vi "Controle_Manip_Main_GUI_Backup2.vi"() -> ()   [LabVIEW 2019] (continued)
                                }
                              }
                              n869 = local read "MasterStop"() -> (w1062:bool)
                            }
                            "Array fPow" <- w1052
                            "Array fPow Pow" <- w1054
                            n870 = Transpose 2D Array(2D array=w1052) -> (transposed array=w1051:i32[][])
                            n871 = property on="CCD 2D Image Main" class="IntGraph (strict)"("Value"=w1051) -> ()  [unwired: 2 in, 2 out]
                          }
                          frame #3 {
                            # "end"
                            n872 = control-ref of="Acquire fPow"() -> (w1194:refnum<vi>)
                            n873 = control-ref of="N Step Power  Diode Current (A)"() -> (w1195:refnum<vi>)
                            n874 = control-ref of="End Power  Diod Current (A)"() -> (w1196:refnum<vi>)
                            n875 = control-ref of="Start Power Diod Current (A)"() -> (w1197:refnum<vi>)
                            n876 = property class="Bool (strict)"(reference=w1194, "Value"=FALSE) -> ()  [unwired: 1 in, 2 out]
                            n877 = control-ref of="Acquire fPow"() -> (w1201:refnum<vi>)
                            n878 = control-ref of="Save fPow"() -> (w1199:refnum<vi>)
                            n879 = Build Array(w1201, w1199, w1197, w1196, w1195) -> (w1200:refnum<vi>[])
                            n880 = call "Enable&Disable_Controls.vi"("Enum"=enum16{"Enabled", "Disabled", "Disabled&Grayed"}."Enabled", "References"=w1200) -> ()  [unwired: 1 in]
                            n881 = property on="Elapsed (s)" class="DigNum (strict)"("Visible"=FALSE) -> ()  [unwired: 2 in, 2 out]
                            n882 = local read "Auto< ?"() -> (w1189:bool)
                            n883 = control-ref of="Save fPow"() -> (w1191:refnum<vi>)
                            n884 = case shown="True" w1189 {
                              tunnel: [TRUE FALSE] -> w1188
                              frame False {
                              }
                              frame True {
                              }
                            }
                            n885 = control-ref of="MasterStop"() -> (w1186:refnum<vi>)
                            n886 = control-ref of="MasterPause"() -> (w1187:refnum<vi>)
                            n887 = control-ref of="ExperimentStopped?"() -> (w1185:refnum<vi>)
                            n888 = call "CheckStopAndReset.vi"("ExperimentStopped?"=w1185, "MasterStop"=w1186, "MasterPause"=w1187) -> ()
                            n889 = control-ref of="Acquire fPow"() -> (w1192:refnum<vi>)
                            n890 = property class="Bool (strict)"(reference=w1192, "Visible"=TRUE) -> ()  [unwired: 1 in, 2 out]
                            n891 = property class="Bool (strict)"(reference=w1191, "Visible"=w1188) -> ()  [unwired: 1 in, 2 out]
                            n892 = property on="CCD 2D Image Main" class="IntGraph (strict)"("Visible"=TRUE) -> ()  [unwired: 2 in, 2 out]
                            n893 = property on="CCD 1D Spectrum Main" class="XYGraph (strict)"("Visible"=FALSE) -> ()  [unwired: 2 in, 2 out]
                          }
                        }
                      }
                      frame "Fast Acq" {
                        n894 = stacked-sequence {
                          frame #0 {
                            w1204 = AcqMode."Spectrum" ("Acq Mode")
                            # "set port to CCD if not already"
                            n895 = property on="Acq Mode" class="Enum (strict)"() -> ("Value"=w1206:T3)  [unwired: 2 in, 2 out]
                            n896 = Not Equal?(x=w1206, y=w1204) -> (x != y?=w1205:bool)
                            n897 = case shown="True" w1205 {
                              tunnel: w1204 -> [_ w1208]
                              frame False {
                              }
                              frame True {
                                w1207 = T33 4 items=["None"=1, "SideEntrance"=2, "FrontEntrance"=3, "SideExit"=5, "FrontExit"=4] ("Exit Port Location")
                                n898 = local read "LightField Automation error out"() -> (w1218:errorcluster)
                                n899 = local read "LightField Automation out"() -> (w1217:refnum<class "LightField Automation.lvclass">)
                                n900 = property on="Acq Mode" class="Enum (strict)"("Value"=w1208) -> ()  [unwired: 2 in, 2 out]
                                n901 = call "spec_SetOpticalExitPort.vi"("error in (no error)"=w1218, "Exit Port Location"=w1207, "LightField Automation in"=w1217) -> ("error out"=w1210:errorcluster, "LightField Automation out"=w1209:refnum<class "LightField Automation.lvclass">)  [unwired: 7 in]
                                n902 = call "spec_GetCenterWavelength.vi"("error in (no error)"=w1210, "LightField Automation in"=w1209) -> ("error out"=w1213:errorcluster, "Center Wavelength"=w1211:dbl, "LightField Automation out"=w1212:refnum<class "LightField Automation.lvclass">)  [unwired: 7 in]
                                n903 = local write "Exit mirror"(w1207) -> ()
                                n904 = local write "Center Wavelength (nm)"(w1211) -> ()
                                n905 = call "spec_getCalibration.vi"("error in (no error)"=w1213, "LightField Automation in"=w1212) -> ("error out"=w1216:errorcluster, "ColumnCalibration"=w1214:dbl[], "LightField Automation out"=w1215:refnum<class "LightField Automation.lvclass">)  [unwired: 7 in]
                                n906 = local write "Wavelength calibration"(w1214) -> ()
                                n907 = local write "LightField Automation error out"(w1216) -> ()
                                n908 = local write "LightField Automation out"(w1215) -> ()
                              }
                            }
                          }
                          frame #1 {
                            # "background if none"
                            n909 = local read "Background taken?"() -> (w1219:bool)
                            n910 = case shown="False" w1219 {
                              frame False {
                                n911 = stacked-sequence {
                                tunnel: [_ _ w1265] -> w1220
                                frame #0 {
                                n912 = property on="CCD 1D Spectrum Main" class="XYGraph (strict)"("YScale.Offset"=0.0 ("Y Scale.Offset and Multiplier:Offset")) -> ()  [unwired: 2 in, 2 out]
                                }
                                frame #1 {
                                # "make sure shutter is closed"
                                n913 = local read "KCube Shutter On?"() -> (w1251:bool)
                                n914 = control-ref of="Shutter Ctrls"() -> (w1255:refnum<vi>)
                                n915 = property class="Ring (strict)"(reference=w1255) -> ("Value"=w1254:u16)  [unwired: 1 in, 2 out]
                                n916 = control-ref of="KCube Shutter Device Reference"() -> (w1256:refnum<vi>)
                                n917 = Equal?(x=w1254, y=u16 0) -> (x = y?=w1252:bool)
                                n918 = case shown="False" w1252 {
                                tunnel: w1256 -> [w1259 _]
                                tunnel: w1255 -> [w1258 _]
                                tunnel: w1251 -> [w1257 _]
                                frame False {
                                n919 = call "Shutter.vi"("KCube Shutter Device Reference 2"=w1259, "Shutter Ctrls 2"=w1258, "Shutter on?"=w1257) -> ()
                                }
                                frame True {
                                }
                                }
                                }
                                frame #2 {
                                # "acquire"
                                n920 = local read "LightField Automation error out"() -> (w1263:errorcluster)
                                n921 = local read "LightField Automation out"() -> (w1264:refnum<class "LightField Automation.lvclass">)
                                n922 = local read "Accumulations"() -> (w1260:dbl)
                                n923 = call "LFA_Capture.vi"("error in (no error)"=w1263, "Frames"=w1260, "LightField Automation in"=w1264) -> ("error out"=w1262:errorcluster, "Data"=w1265:T26, "LightField Automation out"=w1261:refnum<class "LightField Automation.lvclass">)  [unwired: 6 in]
                                n924 = local write "LightField Automation error out"(w1262) -> ()
                                n925 = local write "LightField Automation out"(w1261) -> ()
                                }
                                }
                                n926 = local read "Acq Mode"() -> (w1221:T3)
                                n927 = case shown="\"Spectrum\", Default" w1221 {
                                selector: w1221 -> [w1222 w1240]
                                tunnel: w1220 -> [w1223 w1241]
                                frame "Spectrum", Default {
                                n928 = stacked-sequence {
                                tunnel: w1223 -> [_ w1234 _ _]
                                tunnel: w1222 -> [_ w1232 _ _]
                                frame #0 {
                                n929 = property on="CCD 2D Image Main" class="IntGraph (strict)"("Visible"=FALSE) -> ()  [unwired: 2 in, 2 out]
                                n930 = property on="CCD 1D Spectrum Main" class="XYGraph (strict)"("Visible"=TRUE) -> ()  [unwired: 2 in, 2 out]
                                }
                                frame #1 {
                                n931 = local read "Wavelength calibration"() -> (w1231:dbl[])
                                n932 = local read "CCD ROI"() -> (w1227:T20)
                                n933 = Divide(x=1239.842, y=w1231) -> (x/y=w1229:dbl[])
                                n934 = call "PrepareData4Graph.vi"("Wavelength nm"=w1229, "DataLF"=w1234, "CCD ROI"=w1227, "AcqMode"=w1232, "Data type"=T30."Spectre") -> ("Spectrum"=w1233:cluster{"Array 2":dbl[], "Array":dbl[]}, "PLInt out"=w1226:dbl[])  [unwired: 2 in, 2 out]
                                n935 = local write "CCD 1D Spectrum Main"(w1233) -> ()
                                n936 = local write "BackgroundSpec"(w1226) -> ()
                                }
                                frame #2 {
                                n937 = local read "BackgroundSpec"() -> (w1235:dbl[])
                                n938 = call-poly <vilib>:"Mean.vi"("X"=w1235) -> ("mean"=w1237:dbl)  [unwired: 1 out]
                                n939 = Negate(x=w1237) -> (-x=w1236:dbl)
                                n940 = property on="CCD 1D Spectrum Main" class="XYGraph (strict)"("YScale.Offset"=w1236) -> ()  [unwired: 2 in, 2 out]
                                }
                                frame #3 {
                                n941 = local write "Background taken?"(TRUE ("Background taken?")) -> ()
                                n942 = property on="Background substract" class="Enum (strict)"("Value"=enum16{"None", "Shutter"}."None" ("Background substract")) -> ()  [unwired: 2 in, 2 out]
                                }
                                }
                                }
                                frame "Image" {
                                n943 = stacked-sequence {
                                tunnel: w1241 -> [_ w1249]
                                tunnel: w1240 -> [_ w1247]
                                frame #0 {
                                n944 = property on="CCD 1D Spectrum Main" class="XYGraph (strict)"("Visible"=FALSE) -> ()  [unwired: 2 in, 2 out]
                                n945 = property on="CCD 2D Image Main" class="IntGraph (strict)"("Visible"=TRUE) -> ()  [unwired: 2 in, 2 out]
                                }
                                frame #1 {
                                n946 = local read "Wavelength calibration"() -> (w1248:dbl[])
                                n947 = local read "CCD ROI"() -> (w1244:T20)
                                n948 = call "PrepareData4Graph.vi"("Wavelength nm"=w1248, "DataLF"=w1249, "CCD ROI"=w1244, "AcqMode"=w1247, "Data type"=T30."Spectre") -> ("Intensity Graph"=w1246:dbl[][])  [unwired: 2 in, 3 out]
                                n949 = local write "CCD 2D Image Main"(w1246) -> ()
                                }
                                }
                                }
                                }
                              }
                              frame True {
                              }
                            }
                          }
                          frame #2 {
                            # "\"measurement\""
                            n950 = stacked-sequence {
                              frame #0 {
                                # "open shutter if closed"
                                n951 = control-ref of="Shutter Ctrls"() -> (w1267:refnum<vi>)
                                n952 = property class="Ring (strict)"(reference=w1267) -> ("Value"=w1269:u16)  [unwired: 1 in, 2 out]
                                n953 = local read "KCube Shutter On?"() -> (w1272:bool)
                                n954 = control-ref of="KCube Shutter Device Reference"() -> (w1268:refnum<vi>)
                                n955 = property on="Experiment Graph Controls" class="TabCtl (strict)"("Value"=T25."Spectrum" ("Experiment Graph Controls")) -> ()  [unwired: 2 in, 2 out]
                                n956 = Equal?(x=w1269, y=u16 0) -> (x = y?=w1271:bool)
                                n957 = case shown="True" w1271 {
                                tunnel: w1268 -> [_ w1275]
                                tunnel: w1267 -> [_ w1274]
                                tunnel: w1272 -> [_ w1273]
                                frame False {
                                }
                                frame True {
                                n958 = call "Shutter.vi"("KCube Shutter Device Reference 2"=w1275, "Shutter Ctrls 2"=w1274, "Shutter on?"=w1273) -> ()
                                }
                                }
                              }
                              frame #1 {
                                # "set CCD ROI and acquire"
                                n959 = local read "LightField Automation error out"() -> (w1283:errorcluster)
                                n960 = local read "LightField Automation out"() -> (w1284:refnum<class "LightField Automation.lvclass">)
                                n961 = local read "CCD ROI"() -> (w1282:T20)
                                n962 = local read "Accumulations"() -> (w1279:dbl)
                                n963 = call "Adv_SetROI.vi"("error in (no error)"=w1283, "ROI"=w1282, "LightField Automation in"=w1284) -> ("error out"=w1280:errorcluster, "LightField Automation out"=w1281:refnum<class "LightField Automation.lvclass">)  [unwired: 7 in]
                                n964 = call "LFA_Capture.vi"("error in (no error)"=w1280, "Frames"=w1279, "LightField Automation in"=w1281) -> ("error out"=w1277:errorcluster, "Data"=w1276:T26, "LightField Automation out"=w1278:refnum<class "LightField Automation.lvclass">)  [unwired: 6 in]
                                n965 = local write "LightField Automation out"(w1278) -> ()
                                n966 = local write "LightField Automation error out"(w1277) -> ()
                                n967 = local write "Data"(w1276) -> ()
                              }
                              frame #2 {
                                # "close shutter"
                                n968 = local read "KCube Shutter On?"() -> (w1287:bool)
                                n969 = control-ref of="KCube Shutter Device Reference"() -> (w1286:refnum<vi>)
                                n970 = control-ref of="Shutter Ctrls"() -> (w1285:refnum<vi>)
                                n971 = call "Shutter.vi"("KCube Shutter Device Reference 2"=w1286, "Shutter Ctrls 2"=w1285, "Shutter on?"=w1287) -> ()
                              }
                              frame #3 {
                                # "Show data accordingly"
                                n972 = local read "Acq Mode"() -> (w1289:T3)
                                n973 = local read "Data"() -> (w1288:T26)
                                n974 = case shown="\"Spectrum\", Default" w1289 {
                                selector: w1289 -> [w1290 w1309]
                                tunnel: w1288 -> [w1291 w1310]
                                frame "Spectrum", Default {
                                n975 = stacked-sequence {
                                tunnel: w1291 -> [_ w1307 _]
                                tunnel: w1290 -> [_ w1305 _]
                                frame #0 {
                                n976 = property on="CCD 1D Spectrum Main" class="XYGraph (strict)"("Visible"=TRUE) -> ()  [unwired: 2 in, 2 out]
                                n977 = property on="CCD 2D Image Main" class="IntGraph (strict)"("Visible"=FALSE) -> ()  [unwired: 2 in, 2 out]
                                }
                                frame #1 {
                                n978 = local read "Wavelength calibration"() -> (w1304:dbl[])
                                n979 = local read "CCD ROI"() -> (w1300:T20)
                                n980 = Divide(x=1239.842, y=w1304) -> (x/y=w1302:dbl[])
                                n981 = call "PrepareData4Graph.vi"("Wavelength nm"=w1302, "DataLF"=w1307, "CCD ROI"=w1300, "AcqMode"=w1305, "Data type"=T30."Spectre") -> ("Spectrum"=w1306:cluster{"Array 2":dbl[], "Array":dbl[]}, "PLInt out"=w1299:dbl[])  [unwired: 2 in, 2 out]
                                n982 = local read "Excitation Power (uW)"() -> (w1296:dbl)
                                n983 = local write "CCD 1D Spectrum Main"(w1306) -> ()
                                n984 = local read "Acq Time (ms)"() -> (w1297:dbl)
                                n985 = local read "BackgroundSpec"() -> (w1295:dbl[])
                                n986 = local read "Display Mode"() -> (w1294:u16)
                                n987 = control-ref of="Cnts"() -> (w1298:refnum<vi>)
                                n988 = call "2Cnts.vi"("Array Background"=w1295, "Pow W"=w1296, "AcqTime ms"=w1297, "Cnts Ref"=w1298, "Display Mode"=w1294, "Array"=w1299) -> ()  [unwired: 1 out]
                                }
                                frame #2 {
                                n989 = property on="Full scale" class="Bool (strict)"("Val(Sgnl)"=TRUE ("Value (Signaling)")) -> ()  [unwired: 2 in, 2 out]
                                }
                                }
                                }
                                frame "Image" {
                                n990 = stacked-sequence {
                                tunnel: w1310 -> [_ w1318]
                                tunnel: w1309 -> [_ w1316]
                                frame #0 {
                                n991 = property on="CCD 1D Spectrum Main" class="XYGraph (strict)"("Visible"=FALSE) -> ()  [unwired: 2 in, 2 out]
                                n992 = property on="CCD 2D Image Main" class="IntGraph (strict)"("Visible"=TRUE) -> ()  [unwired: 2 in, 2 out]
                                }
                                frame #1 {
                                n993 = local read "Wavelength calibration"() -> (w1317:dbl[])
                                n994 = local read "CCD ROI"() -> (w1313:T20)
                                n995 = call "PrepareData4Graph.vi"("Wavelength nm"=w1317, "DataLF"=w1318, "CCD ROI"=w1313, "AcqMode"=w1316, "Data type"=T30."Spectre") -> ("Intensity Graph"=w1315:dbl[][])  [unwired: 2 in, 3 out]
                                n996 = local write "CCD 2D Image Main"(w1315) -> ()
                                }
                                }
                                }
                                }
                              }
                            }
                          }
                        }
                      }
                      frame "Acquire Custom Diode Spectrum" {
                        n997 = stacked-sequence {
                          frame #0 {
                            # "change exit slit to APD if needed"
                            n998 = local read "Spectrum Custom Mode"() -> (w1320:u16)
                            n999 = case shown="3" w1320 {
                              frame 0, Default {
                                n1000 = control-ref of="Accumulations"() -> (w1327:refnum<vi>)
                                n1001 = control-ref of="CCD ROI"() -> (w1328:refnum<vi>)
                                n1002 = control-ref of="Exposure Time (ms)"() -> (w1329:refnum<vi>)
                                n1003 = stacked-sequence {
                                tunnel: u16 5 ("NewVal") -> [w1331 w1336 _]
                                tunnel: [_ w1335 _] -> w1325
                                tunnel: [_ w1334 _] -> w1324
                                frame #0 {
                                n1004 = control-ref of="Exit mirror"() -> (w1330:refnum<vi>)
                                n1005 = property class="Ring (strict)"(reference=w1330, "Value"=w1331) -> ()  [unwired: 1 in, 2 out]
                                n1006 = Build Array(w1330) -> (w1333:refnum<vi>[])
                                n1007 = call "Enable&Disable_Controls.vi"("Enum"=enum16{"Enabled", "Disabled", "Disabled&Grayed"}."Disabled&Grayed", "References"=w1333) -> ()  [unwired: 1 in]
                                }
                                frame #1 {
                                n1008 = local read "LightField Automation error out"() -> (w1344:errorcluster)
                                n1009 = case shown="4, Default" w1336 {
                                tunnel: [enum16{"Enabled", "Disabled", "Disabled&Grayed"}."Disabled&Grayed" ("Enum") enum16{"Enabled", "Disabled", "Disabled&Grayed"}."Enabled" ("Enum")] -> w1335
                                tunnel: [AcqMode."APD 1" ("Acq Mode") AcqMode."Spectrum" ("Acq Mode")] -> w1334
                                frame 5 {
                                }
                                frame 4, Default {
                                }
                                }
                                n1010 = local read "LightField Automation out"() -> (w1343:refnum<class "LightField Automation.lvclass">)
                                n1011 = call "spec_GetOpticalExitPort.vi"("error in (no error)"=w1344, "LightField Automation in"=w1343) -> ("error out"=w1341:errorcluster, "Exit Port Location"=w1340:T33, "LightField Automation out"=w1342:refnum<class "LightField Automation.lvclass">)  [unwired: 7 in]
                                n1012 = Equal?(x=w1340, y=w1336) -> (x = y?=w1339:bool)
                                n1013 = case shown="False" w1339 {
                                tunnel: w1342 -> [w1365 w1367]
                                tunnel: w1341 -> [w1364 w1366]
                                tunnel: w1336 -> [w1363 _]
                                tunnel: [w1356 w1367] -> w1338
                                tunnel: [w1355 w1366] -> w1337
                                frame False {
                                n1014 = call "spec_SetOpticalExitPort.vi"("error in (no error)"=w1364, "Exit Port Location"=w1363, "LightField Automation in"=w1365) -> ("error out"=w1358:errorcluster, "LightField Automation out"=w1357:refnum<class "LightField Automation.lvclass">)  [unwired: 7 in]
                                n1015 = call "spec_GetCenterWavelength.vi"("error in (no error)"=w1358, "LightField Automation in"=w1357) -> ("error out"=w1361:errorcluster, "Center Wavelength"=w1359:dbl, "LightField Automation out"=w1360:refnum<class "LightField Automation.lvclass">)  [unwired: 7 in]
                                n1016 = local write "Center Wavelength (nm)"(w1359) -> ()
                                n1017 = call "spec_getCalibration.vi"("error in (no error)"=w1361, "LightField Automation in"=w1360) -> ("error out"=w1355:errorcluster, "ColumnCalibration"=w1362:dbl[], "LightField Automation out"=w1356:refnum<class "LightField Automation.lvclass">)  [unwired: 7 in]
                                n1018 = local write "Wavelength calibration"(w1362) -> ()
                                n1019 = property on="Exit mirror" class="Ring (strict)"() -> ("RingText.Text"=w1351:string)  [unwired: 2 in, 2 out]
                                n1020 = local read "Log file"() -> (w1354:string)
                                n1021 = Concatenate Strings("Exit mirror set to " ("Add to log file"), w1351) -> (w1352:string)
                                n1022 = call "Write2LogFile.vi"("Add to log file"=w1352, "Log file before"=w1354, "Checkbox"=FALSE) -> ("Log file after"=w1353:string)
                                n1023 = local write "Log file"(w1353) -> ()
                                }
                                frame True {
                                }
                                }
                                n1024 = local write "LightField Automation error out"(w1337) -> ()
                                n1025 = local write "LightField Automation out"(w1338) -> ()
                                }
                                frame #2 {
                                n1026 = control-ref of="Exit mirror"() -> (w1370:refnum<vi>)
                                n1027 = Build Array(w1370) -> (w1369:refnum<vi>[])
                                n1028 = call "Enable&Disable_Controls.vi"("Enum"=enum16{"Enabled", "Disabled", "Disabled&Grayed"}."Enabled", "References"=w1369) -> ()  [unwired: 1 in]
                                }
                                }
                                n1029 = Build Array(w1327, w1328, w1329) -> (w1326:refnum<vi>[])
                                n1030 = call "Enable&Disable_Controls.vi"("Enum"=w1325, "References"=w1326) -> ()  [unwired: 1 in]
                                n1031 = property on="Acq Mode" class="Enum (strict)"("Value"=w1324) -> ()  [unwired: 2 in, 2 out]
                              }
                              frame 1 {
                                n1032 = control-ref of="Accumulations"() -> (w1375:refnum<vi>)
                                n1033 = control-ref of="CCD ROI"() -> (w1376:refnum<vi>)
                                n1034 = control-ref of="Exposure Time (ms)"() -> (w1377:refnum<vi>)
                                n1035 = stacked-sequence {
                                tunnel: u16 5 ("NewVal") -> [w1379 w1384 _]
                                tunnel: [_ w1383 _] -> w1373
                                tunnel: [_ w1382 _] -> w1372
                                frame #0 {
                                n1036 = control-ref of="Exit mirror"() -> (w1378:refnum<vi>)
                                n1037 = property class="Ring (strict)"(reference=w1378, "Value"=w1379) -> ()  [unwired: 1 in, 2 out]
                                n1038 = Build Array(w1378) -> (w1381:refnum<vi>[])
                                n1039 = call "Enable&Disable_Controls.vi"("Enum"=enum16{"Enabled", "Disabled", "Disabled&Grayed"}."Disabled&Grayed", "References"=w1381) -> ()  [unwired: 1 in]
                                }
                                frame #1 {
                                n1040 = local read "LightField Automation error out"() -> (w1392:errorcluster)
                                n1041 = case shown="5" w1384 {
                                tunnel: [enum16{"Enabled", "Disabled", "Disabled&Grayed"}."Disabled&Grayed" ("Enum") enum16{"Enabled", "Disabled", "Disabled&Grayed"}."Enabled" ("Enum")] -> w1383
                                tunnel: [AcqMode."APD 1" ("Acq Mode") AcqMode."Spectrum" ("Acq Mode")] -> w1382
                                frame 5 {
                                }
                                frame 4, Default {
                                }
                                }
                                n1042 = local read "LightField Automation out"() -> (w1391:refnum<class "LightField Automation.lvclass">)
                                n1043 = call "spec_GetOpticalExitPort.vi"("error in (no error)"=w1392, "LightField Automation in"=w1391) -> ("error out"=w1389:errorcluster, "Exit Port Location"=w1388:T33, "LightField Automation out"=w1390:refnum<class "LightField Automation.lvclass">)  [unwired: 7 in]
                                n1044 = Equal?(x=w1388, y=w1384) -> (x = y?=w1387:bool)
                                n1045 = case shown="False" w1387 {
                                tunnel: w1390 -> [w1413 w1415]
                                tunnel: w1389 -> [w1412 w1414]
                                tunnel: w1384 -> [w1411 _]
                                tunnel: [w1404 w1415] -> w1386
                                tunnel: [w1403 w1414] -> w1385
                                frame False {
                                n1046 = call "spec_SetOpticalExitPort.vi"("error in (no error)"=w1412, "Exit Port Location"=w1411, "LightField Automation in"=w1413) -> ("error out"=w1406:errorcluster, "LightField Automation out"=w1405:refnum<class "LightField Automation.lvclass">)  [unwired: 7 in]
                                n1047 = call "spec_GetCenterWavelength.vi"("error in (no error)"=w1406, "LightField Automation in"=w1405) -> ("error out"=w1409:errorcluster, "Center Wavelength"=w1407:dbl, "LightField Automation out"=w1408:refnum<class "LightField Automation.lvclass">)  [unwired: 7 in]
                                n1048 = local write "Center Wavelength (nm)"(w1407) -> ()
                                n1049 = call "spec_getCalibration.vi"("error in (no error)"=w1409, "LightField Automation in"=w1408) -> ("error out"=w1403:errorcluster, "ColumnCalibration"=w1410:dbl[], "LightField Automation out"=w1404:refnum<class "LightField Automation.lvclass">)  [unwired: 7 in]
                                n1050 = local write "Wavelength calibration"(w1410) -> ()
                                n1051 = property on="Exit mirror" class="Ring (strict)"() -> ("RingText.Text"=w1399:string)  [unwired: 2 in, 2 out]
                                n1052 = local read "Log file"() -> (w1402:string)
                                n1053 = Concatenate Strings("Exit mirror set to " ("Add to log file"), w1399) -> (w1400:string)
                                n1054 = call "Write2LogFile.vi"("Add to log file"=w1400, "Log file before"=w1402, "Checkbox"=FALSE) -> ("Log file after"=w1401:string)
                                n1055 = local write "Log file"(w1401) -> ()
                                }
                                frame True {
                                }
                                }
                                n1056 = local write "LightField Automation error out"(w1385) -> ()
                                n1057 = local write "LightField Automation out"(w1386) -> ()
                                }
                                frame #2 {
                                n1058 = control-ref of="Exit mirror"() -> (w1418:refnum<vi>)
                                n1059 = Build Array(w1418) -> (w1417:refnum<vi>[])
                                n1060 = call "Enable&Disable_Controls.vi"("Enum"=enum16{"Enabled", "Disabled", "Disabled&Grayed"}."Enabled", "References"=w1417) -> ()  [unwired: 1 in]
                                }
                                }
                                n1061 = Build Array(w1375, w1376, w1377) -> (w1374:refnum<vi>[])
                                n1062 = call "Enable&Disable_Controls.vi"("Enum"=w1373, "References"=w1374) -> ()  [unwired: 1 in]
                                n1063 = property on="Acq Mode" class="Enum (strict)"("Value"=w1372) -> ()  [unwired: 2 in, 2 out]
                              }
                              frame 3 {
                                n1064 = control-ref of="Accumulations"() -> (w1423:refnum<vi>)
                                n1065 = control-ref of="CCD ROI"() -> (w1424:refnum<vi>)
                                n1066 = control-ref of="Exposure Time (ms)"() -> (w1425:refnum<vi>)
                                n1067 = stacked-sequence {
                                tunnel: u16 5 ("NewVal") -> [w1427 w1432 _]
                                tunnel: [_ w1431 _] -> w1421
                                tunnel: [_ w1430 _] -> w1420
                                frame #0 {
                                n1068 = control-ref of="Exit mirror"() -> (w1426:refnum<vi>)
                                n1069 = property class="Ring (strict)"(reference=w1426, "Value"=w1427) -> ()  [unwired: 1 in, 2 out]
                                n1070 = Build Array(w1426) -> (w1429:refnum<vi>[])
                                n1071 = call "Enable&Disable_Controls.vi"("Enum"=enum16{"Enabled", "Disabled", "Disabled&Grayed"}."Disabled&Grayed", "References"=w1429) -> ()  [unwired: 1 in]
                                }
                                frame #1 {
                                n1072 = local read "LightField Automation error out"() -> (w1440:errorcluster)
                                n1073 = case shown="4, Default" w1432 {
                                tunnel: [enum16{"Enabled", "Disabled", "Disabled&Grayed"}."Disabled&Grayed" ("Enum") enum16{"Enabled", "Disabled", "Disabled&Grayed"}."Enabled" ("Enum")] -> w1431
                                tunnel: [AcqMode."APD 1+2" ("Acq Mode") AcqMode."Spectrum" ("Acq Mode")] -> w1430
                                frame 5 {
                                }
                                frame 4, Default {
                                }
                                }
                                n1074 = local read "LightField Automation out"() -> (w1439:refnum<class "LightField Automation.lvclass">)
                                n1075 = call "spec_GetOpticalExitPort.vi"("error in (no error)"=w1440, "LightField Automation in"=w1439) -> ("error out"=w1437:errorcluster, "Exit Port Location"=w1436:T33, "LightField Automation out"=w1438:refnum<class "LightField Automation.lvclass">)  [unwired: 7 in]
                                n1076 = Equal?(x=w1436, y=w1432) -> (x = y?=w1435:bool)
                                n1077 = case shown="False" w1435 {
                                tunnel: w1438 -> [w1461 w1463]
                                tunnel: w1437 -> [w1460 w1462]
                                tunnel: w1432 -> [w1459 _]
                                tunnel: [w1452 w1463] -> w1434
                                tunnel: [w1451 w1462] -> w1433
                                frame False {
                                n1078 = call "spec_SetOpticalExitPort.vi"("error in (no error)"=w1460, "Exit Port Location"=w1459, "LightField Automation in"=w1461) -> ("error out"=w1454:errorcluster, "LightField Automation out"=w1453:refnum<class "LightField Automation.lvclass">)  [unwired: 7 in]
                                n1079 = call "spec_GetCenterWavelength.vi"("error in (no error)"=w1454, "LightField Automation in"=w1453) -> ("error out"=w1457:errorcluster, "Center Wavelength"=w1455:dbl, "LightField Automation out"=w1456:refnum<class "LightField Automation.lvclass">)  [unwired: 7 in]
                                n1080 = local write "Center Wavelength (nm)"(w1455) -> ()
                                n1081 = call "spec_getCalibration.vi"("error in (no error)"=w1457, "LightField Automation in"=w1456) -> ("error out"=w1451:errorcluster, "ColumnCalibration"=w1458:dbl[], "LightField Automation out"=w1452:refnum<class "LightField Automation.lvclass">)  [unwired: 7 in]
                                n1082 = local write "Wavelength calibration"(w1458) -> ()
                                n1083 = property on="Exit mirror" class="Ring (strict)"() -> ("RingText.Text"=w1447:string)  [unwired: 2 in, 2 out]
                                n1084 = local read "Log file"() -> (w1450:string)
                                n1085 = Concatenate Strings("Exit mirror set to " ("Add to log file"), w1447) -> (w1448:string)
                                n1086 = call "Write2LogFile.vi"("Add to log file"=w1448, "Log file before"=w1450, "Checkbox"=FALSE) -> ("Log file after"=w1449:string)
                                n1087 = local write "Log file"(w1449) -> ()
                                }
                                frame True {
                                }
                                }
                                n1088 = local write "LightField Automation error out"(w1433) -> ()
                                n1089 = local write "LightField Automation out"(w1434) -> ()
                                }
                                frame #2 {
                                n1090 = control-ref of="Exit mirror"() -> (w1466:refnum<vi>)
                                n1091 = Build Array(w1466) -> (w1465:refnum<vi>[])
                                n1092 = call "Enable&Disable_Controls.vi"("Enum"=enum16{"Enabled", "Disabled", "Disabled&Grayed"}."Enabled", "References"=w1465) -> ()  [unwired: 1 in]
                                }
                                }
                                n1093 = Build Array(w1423, w1424, w1425) -> (w1422:refnum<vi>[])
                                n1094 = call "Enable&Disable_Controls.vi"("Enum"=w1421, "References"=w1422) -> ()  [unwired: 1 in]
                                n1095 = property on="Acq Mode" class="Enum (strict)"("Value"=w1420) -> ()  [unwired: 2 in, 2 out]
                              }
                              frame 2 {
                                n1096 = property on="Acq Mode" class="Enum (strict)"("Value"=AcqMode."APD 2" ("Acq Mode")) -> ()  [unwired: 2 in, 2 out]
                              }
                              frame 4 {
                                n1097 = property on="Acq Mode" class="Enum (strict)"("Value"=AcqMode."APD 2" ("Acq Mode")) -> ()  [unwired: 2 in, 2 out]
                              }
                            }
                            n1098 = local read "Scan Spectrum Cust Params"() -> (w1322:refnum<vi>[])
                            n1099 = call "Enable&Disable_Controls.vi"("Enum"=enum16{"Enabled", "Disabled", "Disabled&Grayed"}."Disabled&Grayed", "References"=w1322) -> ()  [unwired: 1 in]
                            n1100 = property on="Experiment Graph Controls" class="TabCtl (strict)"("Value"=T25."Spectrum" ("Experiment Graph Controls")) -> ()  [unwired: 2 in, 2 out]
                          }
                          frame #1 {
                            n1101 = local read "Spectrum Step Wavelength (nm)"() -> (w1476:dbl)
                            n1102 = local read "Spectrum End Wavelength (nm)"() -> (w1475:dbl)
                            n1103 = local read "Spectrum Start Wavelength (nm)"() -> (w1477:dbl)
                            n1104 = local read "Spectrum Custom Mode"() -> (w1474:u16)
                            n1105 = local read "KCube Shutter On?"() -> (w1473:bool)
                            n1106 = local read "Acq Time (ms)"() -> (w1472:dbl)
                            n1107 = Bundle("Acq Time (ms)"=w1472, "Spectrum Start Wavelength (nm)"=w1477, "Spectrum Step Wavelength (nm)"=w1476, "Spectrum End Wavelength (nm)"=w1475, "Spectrum Custom Mode"=w1474, "KCube Shutter On?"=w1473) -> (→"Scan Spectrum Cust Exp Params":T18)  [unwired: 1 in]
                            n1108 = control-ref of="MasterStop"() -> (w1470:refnum<vi>)
                            n1109 = property class="Bool (strict)"(reference=w1470, "Visible"=TRUE) -> ()  [unwired: 1 in, 2 out]
                          }
                          frame #2 {
                            n1110 = local read "Spectrum Custom Mode"() -> (w1478:u16)
                            n1111 = case shown="1" w1478 {
                              frame 0, Default {
                                # "PD1 \nScan monochromator SpectraPro HRS with photodiode at APD exit slit"
                                n1112 = control-ref of="Scan Main Progess Bar"() -> (w1482:refnum<vi>)
                                n1113 = local read "LightField Automation out"() -> (w1494:refnum<class "LightField Automation.lvclass">)
                                n1114 = local read "Photodiode handle out"() -> (w1493:refnum<visa-resource-name>)
                                n1115 = local read "LightField Automation error out"() -> (w1491:errorcluster)
                                n1116 = local read "Photodiode error out"() -> (w1492:errorcluster)
                                n1117 = control-ref of="CCD 1D Spectrum Main"() -> (w1490:refnum<vi>)
                                n1118 = control-ref of="Center Wavelength (nm)"() -> (w1488:refnum<vi>)
                                n1119 = control-ref of="Stop Spectrum Custom"() -> ()  [unwired: 1 out]
                                n1120 = control-ref of="Excitation Power (uW)"() -> (w1483:refnum<vi>)
                                n1121 = local read "Scan Spectrum Cust Exp Params"() -> (w1489:T18)
                                n1122 = control-ref of="MasterStop"() -> (w1479:refnum<vi>)
                                n1123 = call "CustomSpectrum.vi"("LightField Automation"=w1494, "Photodiode handle out"=w1493, "Stop Spectrum Custom"=w1479, "Photodiode error out"=w1492, "LightField Automation error"=w1491, "CCD 1D Spectrum Main"=w1490, "Center Wavelength (nm)"=w1488, "Scan Spectrum Progess Bar"=w1482, "Excitation Power (uW)"=w1483, "Scan Spectrum Cust Exp Params 2"=w1489) -> ("WLs"=w1481:dbl[], "PL"=w1480:dbl[], "LFA Out"=w1487:refnum<class "LightField Automation.lvclass">, "PD Out"=w1486:refnum<visa-resource-name>, "PD Error Our"=w1485:errorcluster, "LFA Error Out"=w1484:errorcluster)  [unwired: 3 in, 1 out]
                                n1124 = local write "Data PL Custom Diode Spectrum"(w1480) -> ()
                                n1125 = local write "Wavelength calibration"(w1481) -> ()
                                n1126 = local write "LightField Automation out"(w1487) -> ()
                                n1127 = local write "Photodiode handle out"(w1486) -> ()
                                n1128 = local write "LightField Automation error out"(w1484) -> ()
                                n1129 = local write "Photodiode error out"(w1485) -> ()
                              }
                              frame 1 {
                                # "APD1 Scan monochromator SpectraPro HRS and acquire APD 1"
                                n1130 = stacked-sequence {
                                frame #0 {
                                n1131 = property on="Save Custom Diode Spectrum" class="Bool (strict)"("Visible"=FALSE) -> ()  [unwired: 2 in, 2 out]
                                n1132 = local read "KCube Shutter On?"() -> (w1499:bool)
                                n1133 = control-ref of="Shutter Ctrls"() -> (w1500:refnum<vi>)
                                n1134 = control-ref of="KCube Shutter Device Reference"() -> (w1501:refnum<vi>)
                                n1135 = call "Shutter.vi"("KCube Shutter Device Reference 2"=w1501, "Shutter Ctrls 2"=w1500, "Shutter on?"=w1499) -> ()
                                n1136 = property on="CCD 1D Spectrum Main" class="XYGraph (strict)"("YScale.Offset"=0.0 ("Y Scale.Offset and Multiplier:Offset"), "YScale.Minimum"=0.0 ("Y Scale.Range:Minimum")) -> ()  [unwired: 2 in, 2 out]
                                n1137 = property on="Elapsed (s)" class="DigNum (strict)"("Visible"=TRUE) -> ()  [unwired: 2 in, 2 out]
                                }
                                frame #1 {
                                n1138 = local read "PH_Init_Data"() -> (w1513:T11)
                                n1139 = local read "PH_Settings_Params"() -> (w1512:T10)
                                n1140 = Unbundle By Name(w1513) -> ("Deviceindex"=w1510:i32)
                                n1141 = local read "PH_CFD1 level"() -> (w1507:i32)
                                n1142 = local read "PH_CFD1 zero X"() -> (w1506:i32)
                                n1143 = local read "Acq Time (ms)"() -> (w1503:dbl)
                                n1144 = local read "PH_Range No."() -> (w1505:i32)
                                n1145 = local read "PH_CFD0 level"() -> (w1509:i32)
                                n1146 = local read "PH_CFD0 zero X"() -> (w1508:i32)
                                n1147 = local read "PH_SyncDiv"() -> (w1511:enum16{"1", "2", "4", "8"})
                                n1148 = Bundle By Name(cluster=w1512, "SyncDiv"=w1511, "DeviceIndex"=w1510, "CFD0 level"=w1509, "CFD0 zero X"=w1508, "CFD1 level"=w1507, "CFD1 zero X"=w1506, "Range No."=w1505, "StopOnOverflow"=TRUE, "AcqTime (ms)"=w1503) -> (w1502:T10)
                                n1149 = local write "PH_Settings_Params"(w1502) -> ()
                                }
                                frame #2 {
                                n1150 = local read "LightField Automation error out"() -> (w1522:errorcluster)
                                n1151 = local read "Scan Spectrum Cust Exp Params"() -> (w1521:T18)
                                n1152 = control-ref of="Center Wavelength (nm)"() -> (w1524:refnum<vi>)
                                n1153 = control-ref of="CCD 1D Spectrum Main"() -> (w1525:refnum<vi>)
                                n1154 = local read "LightField Automation out"() -> (w1523:refnum<class "LightField Automation.lvclass">)
                                n1155 = local read "PH_Settings_Params"() -> (w1519:T10)
                                n1156 = local read "PH_Init_Data"() -> (w1520:T11)
                                n1157 = control-ref of="Stop Spectrum Custom"() -> ()  [unwired: 1 out]
                                n1158 = control-ref of="Scan Main Progess Bar"() -> (w1526:refnum<vi>)
                                n1159 = control-ref of="MasterStop"() -> (w1514:refnum<vi>)
                                n1160 = call "CustomAPDSpectrum.vi"("LightField Automation"=w1523, "PH_Init_Data"=w1520, "PH_Settings_Params"=w1519, "Stop Spectrum Custom"=w1514, "LightField Automation error"=w1522, "CCD 1D Spectrum Main"=w1525, "Center Wavelength (nm)"=w1524, "Scan Spectrum Progess Bar"=w1526, "Scan Spectrum Cust Exp Params 2"=w1521) -> ("WLs"=w1516:dbl[], "LFA Out"=w1518:refnum<class "LightField Automation.lvclass">, "PL"=→"Data PL Custom Diode Spectrum":dbl[], "LFA Error Out"=w1517:errorcluster)  [unwired: 6 in, 1 out]
                                n1161 = local write "Wavelength calibration"(w1516) -> ()
                                n1162 = local write "LightField Automation error out"(w1517) -> ()
                                n1163 = local write "LightField Automation out"(w1518) -> ()
                                }
                                frame #3 {
                                n1164 = local read "KCube Shutter On?"() -> (w1532:bool)
                                n1165 = control-ref of="Shutter Ctrls"() -> (w1533:refnum<vi>)
                                n1166 = control-ref of="KCube Shutter Device Reference"() -> (w1534:refnum<vi>)
                                n1167 = call "Shutter.vi"("KCube Shutter Device Reference 2"=w1534, "Shutter Ctrls 2"=w1533, "Shutter on?"=w1532) -> ()
                                n1168 = property on="Full scale" class="Bool (strict)"("Val(Sgnl)"=TRUE ("Value (Signaling)")) -> ()  [unwired: 2 in, 2 out]
                                n1169 = property on="Elapsed (s)" class="DigNum (strict)"("Visible"=FALSE) -> ()  [unwired: 2 in, 2 out]
                                n1170 = local write "Background taken?"(FALSE ("Background taken?")) -> ()
                                n1171 = property on="CCD 1D Spectrum Main" class="XYGraph (strict)"("YScale.Offset"=0.0 ("Y Scale.Offset and Multiplier:Offset"), "YScale.Minimum"=0.0 ("Y Scale.Range:Minimum")) -> ()  [unwired: 2 in, 2 out]
                                }
                                }
                              }
                              frame 2 {
                                # "APD2 Scan monochromator iHR320 and acquire APD 2 // quick&dirty avant calib"
                                n1172 = stacked-sequence {
                                frame #0 {
                                w1535 = 0.0 ("Y Scale.Offset and Multiplier:Offset")
                                n1173 = property on="Elapsed (s)" class="DigNum (strict)"("Visible"=TRUE) -> ()  [unwired: 2 in, 2 out]
                                n1174 = property on="Save Custom Diode Spectrum" class="Bool (strict)"("Visible"=FALSE) -> ()  [unwired: 2 in, 2 out]
                                n1175 = local read "KCube Shutter On?"() -> (w1538:bool)
                                n1176 = control-ref of="Shutter Ctrls"() -> (w1539:refnum<vi>)
                                n1177 = control-ref of="KCube Shutter Device Reference"() -> (w1540:refnum<vi>)
                                n1178 = call "Shutter.vi"("KCube Shutter Device Reference 2"=w1540, "Shutter Ctrls 2"=w1539, "Shutter on?"=w1538) -> ()
                                n1179 = property on="CCD 1D Spectrum Main" class="XYGraph (strict)"("YScale.Offset"=w1535, "YScale.Minimum"=w1535) -> ()  [unwired: 2 in, 2 out]
                                }
                                frame #1 {
                                n1180 = local read "PH_Init_Data"() -> (w1551:T11)
                                n1181 = local read "PH_Settings_Params"() -> (w1552:T10)
                                n1182 = Unbundle By Name(w1551) -> ("Deviceindex"=w1549:i32)
                                n1183 = local read "PH_CFD1 level"() -> (w1546:i32)
                                n1184 = local read "PH_CFD1 zero X"() -> (w1545:i32)
                                n1185 = local read "Acq Time (ms)"() -> (w1543:dbl)
                                n1186 = local read "PH_Range No."() -> (w1544:i32)
                                n1187 = local read "PH_CFD0 level"() -> (w1548:i32)
                                n1188 = local read "PH_CFD0 zero X"() -> (w1547:i32)
                                n1189 = local read "PH_SyncDiv"() -> (w1550:enum16{"1", "2", "4", "8"})
                                n1190 = Bundle By Name(cluster=w1552, "SyncDiv"=w1550, "DeviceIndex"=w1549, "CFD0 level"=w1548, "CFD0 zero X"=w1547, "CFD1 level"=w1546, "CFD1 zero X"=w1545, "Range No."=w1544, "StopOnOverflow"=TRUE, "AcqTime (ms)"=w1543) -> (w1542:T10)
                                n1191 = local write "PH_Settings_Params"(w1542) -> ()
                                }
                                frame #2 {
                                n1192 = local read "Spectrum End Wavelength (nm)"() -> (w1560:dbl)
                                n1193 = local read "Spectrum Step Wavelength (nm)"() -> (w1554:dbl)
                                n1194 = local read "Spectrum Start Wavelength (nm)"() -> (w1558:dbl)
                                n1195 = Subtract(x=w1560, y=w1558) -> (x-y=w1562:dbl)
                                n1196 = Divide(x=w1562, y=w1554) -> (x/y=w1561:dbl)
                                n1197 = Increment(x=w1561) -> (x+1=w1559:dbl)
                                n1198 = for {
                                N: w1559 -> [_]
                                tunnel: w1554 -> [w1577]
                                tunnel: w1558 -> [w1576]
                                shift-right: [w1563] -> w1555
                                shift-left: dbl[] [] -> [w1571]
                                shift-right: [w1568] -> w1553
                                shift-left: dbl[] [] -> [w1572]
                                i -> [w1578]
                                stop <- w1566 stop-if-true
                                n1199 = control-ref of="MasterStop"() -> (w1565:refnum<vi>)
                                n1200 = control-ref of="Stop Spectrum Custom"() -> ()  [unwired: 1 out]
                                n1201 = Multiply(x=w1578, y=w1577) -> (x*y=w1575:dbl)
                                n1202 = Add(x=w1576, y=w1575) -> (x+y=w1567:dbl)
                                n1203 = local read "ESP300 COM Port"() -> (w1574:refnum<visa-resource-name>)
                                n1204 = stacked-sequence {
                                tunnel: w1567 -> [w1580 _ _]
                                tunnel: w1574 -> [w1588 _ _]
                                tunnel: [_ _ w1590] -> w1573
                                tunnel: w1572 -> [w1586 _ _]
                                tunnel: [w1585 _ _] -> w1568
                                frame #0 {
                                w1582 = u16 1 items=["Detection"=1, "Excitation"=2] ("HR mode")
                                n1205 = call "MotorWL2Pos.vi"("Mono2 Center WL"=w1580, "HR mode"=w1582) -> ("Mono2 Position"=w1584:dbl)
                                n1206 = control-ref of="Mono2 Motor Pos"() -> (w1587:refnum<vi>)
                                n1207 = control-ref of="Mono2 Wavelength (nm)"() -> (w1583:refnum<vi>)
                                n1208 = call "subVI_Mono2Go2Posv2.vi"("Mono2 Motor Pos"=w1587, "Mono2 Wavelength (nm)"=w1583, "HR mode"=w1582, "Postion (Unit)"=w1584, "ESP300 COM Port"=w1588) -> ()  [unwired: 2 out]
                                n1209 = Divide(x=1239.842, y=w1580) -> (x/y=w1579:dbl)
                                n1210 = Insert Into Array(array=w1586, new element=w1579) -> (w1585:dbl[])  [unwired: 1 in]
                                }
                                frame #1 {
                                n1211 = Wait (ms)(milliseconds to wait=u32 20) -> ()  [unwired: 1 out]
                                }
                                frame #2 {
                                n1212 = local read "PH_Settings_Params"() -> (w1591:T10)
                                n1213 = local read "PH_Init_Data"() -> (w1592:T11)
                                n1214 = Unbundle By Name(w1592) -> ("Initialization Error"=w1596:bool, "Calib Error"=w1595:bool, "Deviceindex"=w1594:i32)
                                n1215 = call "PH_Acq_ms.vi"("PH_Settings_Params"=w1591, "Deviceindex"=w1594, "Calib Error"=w1595, "Initialization Error"=w1596) -> ("CH1MeanRate"=w1590:dbl, "SyncMeanRate"=w1593:dbl)  [unwired: 1 out]
                                n1216 = Build Array(w1593, w1590) -> ()  [unwired: 1 out]
                                }
                                }
                                n1217 = property class="Bool (strict)"(reference=w1565) -> ("Value"=w1566:bool)  [unwired: 1 in, 2 out]
                                n1218 = control-ref of="CCD 1D Spectrum Main"() -> (w1570:refnum<vi>)
                                n1219 = Insert Into Array(array=w1571, new element=w1573) -> (w1563:dbl[])  [unwired: 1 in]
                                n1220 = call "myMaxAPDs.vi"("Array"=w1563) -> ("myMax"=w1564:dbl)
                                n1221 = Bundle(w1568, w1563) -> (w1569:cluster{dbl[], dbl[]})  [unwired: 1 in]
                                n1222 = property class="XYGraph (strict)"(reference=w1570, "Value"=w1569, "YScale.Maximum"=w1564) -> ()  [unwired: 1 in, 2 out]
                                }
                                n1223 = local write "Wavelength calibration"(w1553) -> ()
                                n1224 = local write "Data PL Custom Diode Spectrum"(w1555) -> ()
                                }
                                frame #3 {
                                n1225 = property on="Elapsed (s)" class="DigNum (strict)"("Visible"=FALSE) -> ()  [unwired: 2 in, 2 out]
                                n1226 = local read "KCube Shutter On?"() -> (w1602:bool)
                                n1227 = control-ref of="Shutter Ctrls"() -> (w1603:refnum<vi>)
                                n1228 = property on="CCD 1D Spectrum Main" class="XYGraph (strict)"("YScale.Offset"=0.0 ("Y Scale.Offset and Multiplier:Offset"), "YScale.Minimum"=0.0 ("Y Scale.Range:Minimum")) -> ()  [unwired: 2 in, 2 out]
                                n1229 = control-ref of="KCube Shutter Device Reference"() -> (w1604:refnum<vi>)
                                n1230 = call "Shutter.vi"("KCube Shutter Device Reference 2"=w1604, "Shutter Ctrls 2"=w1603, "Shutter on?"=w1602) -> ()
                                n1231 = local write "Background taken?"(FALSE ("Background taken?")) -> ()
                                n1232 = property on="Full scale" class="Bool (strict)"("Val(Sgnl)"=TRUE ("Value (Signaling)")) -> ()  [unwired: 2 in, 2 out]
                                }
                                }
                              }
                              frame 3 {
                                # "ADP1&2 Scan both monochromators synchronously and both APD outputs"
                              }
                              frame 4 {
                                # "PD2 Scan monochromator iHR320 with photodiode at APD exit slit"
                                n1233 = stacked-sequence {
                                frame #0 {
                                n1234 = property on="Elapsed (s)" class="DigNum (strict)"("Visible"=TRUE) -> ()  [unwired: 2 in, 2 out]
                                n1235 = property on="Save Custom Diode Spectrum" class="Bool (strict)"("Visible"=FALSE) -> ()  [unwired: 2 in, 2 out]
                                n1236 = local read "KCube Shutter On?"() -> (w1607:bool)
                                n1237 = control-ref of="Shutter Ctrls"() -> (w1608:refnum<vi>)
                                n1238 = control-ref of="KCube Shutter Device Reference"() -> (w1609:refnum<vi>)
                                n1239 = call "Shutter.vi"("KCube Shutter Device Reference 2"=w1609, "Shutter Ctrls 2"=w1608, "Shutter on?"=w1607) -> ()
                                }
                                frame #1 {
                                n1240 = local read "PH_Init_Data"() -> (w1620:T11)
                                n1241 = local read "PH_Settings_Params"() -> (w1621:T10)
                                n1242 = local read "PH_CFD1 level"() -> (w1615:i32)
                                n1243 = local read "PH_CFD1 zero X"() -> (w1614:i32)
                                n1244 = local read "Acq Time (ms)"() -> (w1612:dbl)
                                n1245 = local read "PH_Range No."() -> (w1613:i32)
                                n1246 = Unbundle By Name(w1620) -> ("Deviceindex"=w1618:i32)
                                n1247 = local read "PH_CFD0 level"() -> (w1617:i32)
                                n1248 = local read "PH_CFD0 zero X"() -> (w1616:i32)
                                n1249 = local read "PH_SyncDiv"() -> (w1619:enum16{"1", "2", "4", "8"})
                                n1250 = Bundle By Name(cluster=w1621, "SyncDiv"=w1619, "DeviceIndex"=w1618, "CFD0 level"=w1617, "CFD0 zero X"=w1616, "CFD1 level"=w1615, "CFD1 zero X"=w1614, "Range No."=w1613, "StopOnOverflow"=TRUE, "AcqTime (ms)"=w1612) -> (w1611:T10)